vi "FlexMag - 23-03-2023.vi"() -> ()   [LabVIEW 2018] (continued)
                                n14725 = local write "pcgv4 auto open"(TRUE ("pcgv1 auto open")) -> ()
                                }
                                }
                              }
                            }
                          }
                          frame #1 {
                            n14726 = while {
                              i -> [w19971]
                              stop <- w19967 stop-if-true
                              n14727 = Greater Or Equal?(x=w19971, y=200) -> (x >= y?=w19973:bool)
                              n14728 = case shown="True" w19973 {
                                frame False {
                                }
                                frame True {
                                n14729 = local write "ch4 pumpdown error"(TRUE ("ch1 pumpdown error")) -> ()
                                n14730 = local write "Warning Message"("CH4 PumpDown process  is canceled !\nCH4 PC GV couldn't be opened" ("Warning Message")) -> ()
                                }
                              }
                              n14731 = local read "ch4 pumpdown alg"() -> (w19970:bool)
                              n14732 = local read "ch4_pcgv_gui"() -> (w19966:bool)
                              n14733 = local read "abort ch4"() -> (w19968:bool)
                              n14734 = Wait Until Next ms Multiple(millisecond multiple=u32 200) -> ()  [unwired: 1 out]
                              n14735 = Not(x=w19970) -> (.not. x?=w19969:bool)
                              n14736 = Compound Arithmetic op=OR(w19966, w19968, w19969) -> (w19967:bool)
                            }
                          }
                        }
                      }
                      frame True {
                      }
                    }
                  }
                }
              }
              frame #20 {
                n14737 = local read "ch4 pumpdown alg"() -> (w19976:bool)
                n14738 = case shown="True" w19976 {
                  frame False {
                  }
                  frame True {
                    n14739 = local read "abort ch4"() -> (w19977:bool)
                    n14740 = case shown="False" w19977 {
                      frame False {
                        n14741 = local write "ch4 pc gv open led"(TRUE ("ch1 ch vbv close")) -> ()
                        n14742 = Wait (ms)(milliseconds to wait=u32 1000) -> ()  [unwired: 1 out]
                      }
                      frame True {
                      }
                    }
                  }
                }
              }
              frame #21 {
                # "ch pressure check"
                n14743 = local read "ch4 pumpdown alg"() -> (w19980:bool)
                n14744 = case shown="True" w19980 {
                  frame False {
                  }
                  frame True {
                    n14745 = local read "abort ch4"() -> (w19981:bool)
                    n14746 = case shown="False" w19981 {
                      frame False {
                        n14747 = while {
                          i -> [w19988]
                          stop <- w19992 stop-if-true
                          # "30 min"
                          n14748 = Greater?(x=w19988, y=9000) -> (0:w19985:bool)
                          n14749 = case shown="True" w19985 {
                            frame False {
                            }
                            frame True {
                              n14750 = local write "Warning Message"("CH4 PumpDown process  is canceled !\nCH4 CH Pressure couldn't reach under 0.5 Torr" ("Warning Message")) -> ()
                              n14751 = local write "ch4 pumpdown error"(TRUE ("ch1 pumpdown error")) -> ()
                            }
                          }
                          n14752 = local read "ch4 ch pg torr"() -> (w19984:dbl)
                          n14753 = Less Or Equal?(x=w19984, y=0.5) -> (x <= y?=w19982:bool)
                          n14754 = case shown="False" w19982 {
                            tunnel: [FALSE TRUE] -> w19986
                            frame False {
                              n14755 = Wait Until Next ms Multiple(millisecond multiple=u32 200) -> ()  [unwired: 1 out]
                            }
                            frame True {
                            }
                          }
                          n14756 = local read "ch4 pumpdown alg"() -> (w19991:bool)
                          n14757 = local read "abort ch4"() -> (w19989:bool)
                          n14758 = Not(x=w19991) -> (.not. x?=w19990:bool)
                          n14759 = Compound Arithmetic op=OR(w19986, w19989, w19990) -> (w19992:bool)
                        }
                      }
                      frame True {
                      }
                    }
                  }
                }
              }
              frame #22 {
                n14760 = local read "ch4 pumpdown alg"() -> (w19998:bool)
                n14761 = case shown="True" w19998 {
                  frame False {
                  }
                  frame True {
                    n14762 = local read "abort ch4"() -> (w19999:bool)
                    n14763 = case shown="False" w19999 {
                      frame False {
                        n14764 = local write "ch4 ch press under 0.5 T led"(TRUE ("ch1 ch pressure led")) -> ()
                        n14765 = Wait (ms)(milliseconds to wait=u32 1000) -> ()  [unwired: 1 out]
                      }
                      frame True {
                      }
                    }
                  }
                }
              }
              frame #23 {
                # "ch 3 pressure check\nfor trns bp bv"
                n14766 = local read "ch4 pumpdown alg"() -> (w20002:bool)
                n14767 = case shown="True" w20002 {
                  frame False {
                  }
                  frame True {
                    n14768 = local read "abort ch4"() -> (w20003:bool)
                    n14769 = case shown="False" w20003 {
                      frame False {
                        n14770 = local read "ch3 ch pg torr"() -> (w20006:dbl)
                        n14771 = Less Or Equal?(x=w20006, y=0.5) -> (x <= y?=w20004:bool)
                        n14772 = case shown="True" w20004 {
                          frame False {
                          }
                          frame True {
                            n14773 = stacked-sequence {
                              frame #0 {
                                n14774 = while {
                                i -> [w20011]
                                stop <- w20015 stop-if-true
                                n14775 = Greater?(x=w20011, y=100) -> (0:w20008:bool)
                                n14776 = case shown="True" w20008 {
                                frame False {
                                }
                                frame True {
                                n14777 = local write "ch4 pumpdown error"(TRUE ("ch1 pumpdown error")) -> ()
                                n14778 = local write "Warning Message"("CH4 PumpDown process  is canceled !\nCH4 Trns BP Right couldn't be opened" ("Warning Message")) -> ()
                                }
                                }
                                n14779 = local read "CH4_Trns_BP_Right_DI"() -> (w20007:bool)
                                n14780 = case shown="False" w20007 {
                                tunnel: [FALSE TRUE] -> w20009
                                frame False {
                                n14781 = local write "CH4_Trns_BP_Right_DO"(TRUE ("CH1_Trns_BP_Left_DO")) -> ()
                                n14782 = Wait Until Next ms Multiple(millisecond multiple=u32 200) -> ()  [unwired: 1 out]
                                }
                                frame True {
                                }
                                }
                                n14783 = local read "ch4 pumpdown alg"() -> (w20014:bool)
                                n14784 = local read "abort ch4"() -> (w20012:bool)
                                n14785 = Not(x=w20014) -> (.not. x?=w20013:bool)
                                n14786 = Compound Arithmetic op=OR(w20009, w20012, w20013) -> (w20015:bool)
                                }
                              }
                              frame #1 {
                                n14787 = local read "ch4 pumpdown alg"() -> (w20022:bool)
                                n14788 = case shown="True" w20022 {
                                frame False {
                                }
                                frame True {
                                n14789 = local read "abort ch4"() -> (w20023:bool)
                                n14790 = case shown="False" w20023 {
                                frame False {
                                n14791 = local write "ch4 trns bp right open led"(TRUE ("ch1 tp start led")) -> ()
                                n14792 = Wait (ms)(milliseconds to wait=u32 1000) -> ()  [unwired: 1 out]
                                n14793 = local write "ch3_4 vacuum level"("VACUUM" ("ch3_4 vacuum level")) -> ()
                                }
                                frame True {
                                }
                                }
                                }
                                }
                              }
                              frame #2 {
                                n14794 = while {
                                i -> [w20029]
                                stop <- w20031 stop-if-true
                                n14795 = local read "ch4 pumpdown alg"() -> (w20032:bool)
                                n14796 = Wait Until Next ms Multiple(millisecond multiple=u32 200) -> ()  [unwired: 1 out]
                                n14797 = local read "abort ch4"() -> (w20034:bool)
                                n14798 = Greater?(x=w20029, y=100) -> (0:w20028:bool)
                                n14799 = Not(x=w20032) -> (.not. x?=w20033:bool)
                                n14800 = Compound Arithmetic op=OR(w20028, w20034, w20033) -> (w20031:bool)
                                }
                              }
                            }
                          }
                        }
                      }
                      frame True {
                      }
                    }
                  }
                }
              }
              frame #24 {
                # "ch pressure check"
                n14801 = local read "ch4 pumpdown alg"() -> (w20035:bool)
                n14802 = case shown="True" w20035 {
                  frame False {
                  }
                  frame True {
                    n14803 = local read "abort ch4"() -> (w20036:bool)
                    n14804 = case shown="False" w20036 {
                      frame False {
                        n14805 = while {
                          i -> [w20043]
                          stop <- w20047 stop-if-true
                          # "20 min"
                          n14806 = Greater?(x=w20043, y=6000) -> (0:w20040:bool)
                          n14807 = case shown="True" w20040 {
                            frame False {
                            }
                            frame True {
                              n14808 = local write "Warning Message"("CH4 PumpDown process  is canceled !\nCH4 CH Pressure couldn't  reach under 0.2 Torr" ("Warning Message")) -> ()
                              n14809 = local write "ch4 pumpdown error"(TRUE ("ch1 pumpdown error")) -> ()
                            }
                          }
                          n14810 = local read "ch4 ch pg torr"() -> (w20039:dbl)
                          n14811 = Less Or Equal?(x=w20039, y=0.2) -> (x <= y?=w20037:bool)
                          n14812 = case shown="True" w20037 {
                            tunnel: [FALSE TRUE] -> w20041
                            frame False {
                              n14813 = Wait Until Next ms Multiple(millisecond multiple=u32 200) -> ()  [unwired: 1 out]
                            }
                            frame True {
                            }
                          }
                          n14814 = local read "ch4 pumpdown alg"() -> (w20046:bool)
                          n14815 = local read "abort ch4"() -> (w20044:bool)
                          n14816 = Not(x=w20046) -> (.not. x?=w20045:bool)
                          n14817 = Compound Arithmetic op=OR(w20041, w20044, w20045) -> (w20047:bool)
                        }
                      }
                      frame True {
                      }
                    }
                  }
                }
              }
              frame #25 {
                # "tp start"
                n14818 = local read "ch4 pumpdown alg"() -> (w20053:bool)
                n14819 = case shown="True" w20053 {
                  frame False {
                  }
                  frame True {
                    n14820 = local read "abort ch4"() -> (w20054:bool)
                    n14821 = case shown="False" w20054 {
                      frame False {
                        n14822 = stacked-sequence {
                          frame #0 {
                            n14823 = flat-sequence {
                              frame #0 {
                                n14824 = local write "Tp4 auto start"(TRUE ("Tp1 auto start")) -> ()
                                n14825 = Wait (ms)(milliseconds to wait=u32 100) -> ()  [unwired: 1 out]
                              }
                              frame #1 {
                                n14826 = Wait (ms)(milliseconds to wait=u32 2000) -> ()  [unwired: 1 out]
                              }
                              frame #2 {
                                n14827 = disable-structure shown="Disabled" {
                                frame Disabled {
                                n14828 = local write "Tp1 Start initial"(TRUE ("Tp1 Start initial")) -> ()
                                }
                                frame Enabled {
                                }
                                }
                              }
                              frame #3 {
                                n14829 = Wait (ms)(milliseconds to wait=u32 2000) -> ()  [unwired: 1 out]
                              }
                              frame #4 {
                                n14830 = local write "Tp4 auto low speed"(TRUE ("Tp1 auto start")) -> ()
                                n14831 = Wait (ms)(milliseconds to wait=u32 100) -> ()  [unwired: 1 out]
                              }
                            }
                          }
                          frame #1 {
                            n14832 = while {
                              i -> [w20070]
                              stop <- w20064 stop-if-true
                              # "200 sec ?"
                              n14833 = Greater Or Equal?(x=w20070, y=1000) -> (x >= y?=w20063:bool)
                              n14834 = case shown="True" w20063 {
                                frame False {
                                }
                                frame True {
                                n14835 = local write "Warning Message"("CH4 PumpDown process  is canceled !\nCH4 TP couldn't be started" ("Warning Message")) -> ()
                                n14836 = local write "ch4 pumpdown error"(TRUE ("ch1 pumpdown error")) -> ()
                                }
                              }
                              n14837 = local read "ch4 pumpdown alg"() -> (w20067:bool)
                              n14838 = local read "ch4_tp_gui"() -> (w20062:bool)
                              n14839 = local read "abort ch4"() -> (w20065:bool)
                              n14840 = Not(x=w20067) -> (.not. x?=w20066:bool)
                              n14841 = Wait Until Next ms Multiple(millisecond multiple=u32 200) -> ()  [unwired: 1 out]
                              n14842 = Compound Arithmetic op=OR(w20062, w20065, w20066) -> (w20064:bool)
                            }
                          }
                        }
                      }
                      frame True {
                      }
                    }
                  }
                }
              }
              frame #26 {
                n14843 = local read "ch4 pumpdown alg"() -> (w20073:bool)
                n14844 = case shown="True" w20073 {
                  frame False {
                  }
                  frame True {
                    n14845 = local read "abort ch4"() -> (w20074:bool)
                    n14846 = case shown="False" w20074 {
                      frame False {
                        n14847 = local write "ch4 tp start led"(TRUE ("ch1 tp start led")) -> ()
                        n14848 = Wait (ms)(milliseconds to wait=u32 1000) -> ()  [unwired: 1 out]
                      }
                      frame True {
                      }
                    }
                  }
                }
              }
              frame #27 {
                n14849 = local read "ch4 pumpdown alg"() -> (w20077:bool)
                n14850 = case shown="True" w20077 {
                  frame False {
                  }
                  frame True {
                    n14851 = local read "abort ch4"() -> (w20078:bool)
                    n14852 = case shown="False" w20078 {
                      frame False {
                        n14853 = while {
                          i -> [w20085]
                          stop <- w20089 stop-if-true
                          # "30 min"
                          n14854 = Greater?(x=w20085, y=9000) -> (0:w20082:bool)
                          n14855 = case shown="True" w20082 {
                            frame False {
                            }
                            frame True {
                              n14856 = local write "Warning Message"("CH4 PumpDown process  is canceled !\nCH4 CH Pressure couldn't be reached under 0.01 Torr" ("Warning Message")) -> ()
                              n14857 = local write "ch4 pumpdown error"(TRUE ("ch1 pumpdown error")) -> ()
                            }
                          }
                          n14858 = local read "ch4 ch pg torr"() -> (w20081:dbl)
                          n14859 = Less Or Equal?(x=w20081, y=0.09) -> (x <= y?=w20079:bool)
                          n14860 = case shown="False" w20079 {
                            tunnel: [FALSE TRUE] -> w20083
                            frame False {
                              n14861 = Wait Until Next ms Multiple(millisecond multiple=u32 200) -> ()  [unwired: 1 out]
                            }
                            frame True {
                            }
                          }
                          n14862 = local read "ch4 pumpdown alg"() -> (w20088:bool)
                          n14863 = local read "abort ch4"() -> (w20086:bool)
                          n14864 = Not(x=w20088) -> (.not. x?=w20087:bool)
                          n14865 = Compound Arithmetic op=OR(w20083, w20086, w20087) -> (w20089:bool)
                        }
                      }
                      frame True {
                      }
                    }
                  }
                }
              }
              frame #28 {
                n14866 = local read "ch4 pumpdown alg"() -> (w20095:bool)
                n14867 = case shown="True" w20095 {
                  frame False {
                  }
                  frame True {
                    n14868 = local read "abort ch4"() -> (w20096:bool)
                    n14869 = case shown="False" w20096 {
                      frame False {
                        n14870 = local write "ch4 ch press under 0.01 T led"(TRUE ("ch1 pressure under 0.05 torr led")) -> ()
                        n14871 = Wait (ms)(milliseconds to wait=u32 1000) -> ()  [unwired: 1 out]
                      }
                      frame True {
                      }
                    }
                  }
                }
              }
              frame #29 {
                n14872 = local read "ch4 pumpdown alg"() -> (w20099:bool)
                n14873 = case shown="True" w20099 {
                  frame False {
                  }
                  frame True {
                    n14874 = local read "abort ch4"() -> (w20100:bool)
                    n14875 = case shown="False" w20100 {
                      frame False {
                        n14876 = stacked-sequence {
                          frame #0 {
                            n14877 = while {
                              i -> [w20105]
                              stop <- w20109 stop-if-true
                              n14878 = Greater?(x=w20105, y=200) -> (0:w20102:bool)
                              n14879 = case shown="True" w20102 {
                                frame False {
                                }
                                frame True {
                                n14880 = local write "Warning Message"("CH4 PumpDown process  is canceled !\nCH4 CC couldn't be opened" ("Warning Message")) -> ()
                                n14881 = local write "ch4 pumpdown error"(TRUE ("ch1 pumpdown error")) -> ()
                                }
                              }
                              n14882 = local read "CH4_CC_DI"() -> (w20101:bool)
                              n14883 = case shown="False" w20101 {
                                tunnel: [FALSE TRUE] -> w20103
                                frame False {
                                n14884 = Wait Until Next ms Multiple(millisecond multiple=u32 200) -> ()  [unwired: 1 out]
                                n14885 = local write "CH4_CC_DO"(TRUE ("CH1_CC_DO")) -> ()
                                }
                                frame True {
                                }
                              }
                              n14886 = local read "ch4 pumpdown alg"() -> (w20108:bool)
                              n14887 = local read "abort ch4"() -> (w20106:bool)
                              n14888 = Not(x=w20108) -> (.not. x?=w20107:bool)
                              n14889 = Compound Arithmetic op=OR(w20103, w20106, w20107) -> (w20109:bool)
                            }
                          }
                          frame #1 {
                            n14890 = while {
                              i -> [w20118]
                              stop <- w20120 stop-if-true
                              n14891 = local read "ch4 pumpdown alg"() -> (w20121:bool)
                              n14892 = local read "abort ch4"() -> (w20123:bool)
                              n14893 = Greater Or Equal?(x=w20118, y=300) -> (x >= y?=w20116:bool)
                              n14894 = Not(x=w20121) -> (.not. x?=w20122:bool)
                              n14895 = Compound Arithmetic op=OR(w20116, w20123, w20122) -> (w20120:bool)
                              n14896 = Wait Until Next ms Multiple(millisecond multiple=u32 200) -> ()  [unwired: 1 out]
                            }
                          }
                        }
                      }
                      frame True {
                      }
                    }
                  }
                }
              }
              frame #30 {
                n14897 = local read "ch4 pumpdown alg"() -> (w20124:bool)
                n14898 = case shown="True" w20124 {
                  frame False {
                  }
                  frame True {
                    n14899 = local read "abort ch4"() -> (w20125:bool)
                    n14900 = case shown="False" w20125 {
                      frame False {
                        n14901 = local write "ch4 cc open led"(TRUE ("ch1 ch cc open led")) -> ()
                        n14902 = Wait (ms)(milliseconds to wait=u32 1000) -> ()  [unwired: 1 out]
                      }
                      frame True {
                      }
                    }
                  }
                }
              }
              frame #31 {
                n14903 = local read "ch4 pumpdown alg"() -> (w20128:bool)
                n14904 = case shown="True" w20128 {
                  frame False {
                  }
                  frame True {
                    n14905 = local read "abort ch4"() -> (w20129:bool)
                    n14906 = case shown="False" w20129 {
                      frame False {
                        n14907 = while {
                          i -> [w20140]
                          stop <- w20144 stop-if-true
                          # "60 min"
                          n14908 = Multiply(x=27000 ("y"), y=3) -> (x*y=w20130:i32)
                          n14909 = Greater?(x=w20140, y=w20130) -> (0:w20138:bool)
                          n14910 = case shown="True" w20138 {
                            frame False {
                            }
                            frame True {
                              n14911 = local write "Warning Message"("CH4 PumpDown process  is canceled !\nCH4 CH Pressure couldn't reach to desired pressure" ("Warning Message")) -> ()
                              n14912 = local write "ch4 pumpdown error"(TRUE ("ch1 pumpdown error")) -> ()
                            }
                          }
                          n14913 = local read "ch4 cc torr"() -> (w20137:dbl)
                          n14914 = Multiply(x=0.75, y="ch4 desired pressure") -> (x*y=w20135:dbl)
                          n14915 = Less Or Equal?(x=w20137, y=w20135) -> (x <= y?=w20136:bool)
                          n14916 = case shown="True" w20136 {
                            tunnel: [FALSE TRUE] -> w20139
                            frame False {
                              n14917 = Wait Until Next ms Multiple(millisecond multiple=u32 200) -> ()  [unwired: 1 out]
                            }
                            frame True {
                            }
                          }
                          n14918 = local read "ch4 pumpdown alg"() -> (w20143:bool)
                          n14919 = local read "abort ch4"() -> (w20141:bool)
                          n14920 = Not(x=w20143) -> (.not. x?=w20142:bool)
                          n14921 = Compound Arithmetic op=OR(w20139, w20141, w20142) -> (w20144:bool)
                        }
                      }
                      frame True {
                      }
                    }
                  }
                }
              }
              frame #32 {
                n14922 = local read "ch4 pumpdown alg"() -> (w20150:bool)
                n14923 = case shown="True" w20150 {
                  frame False {
                  }
                  frame True {
                    n14924 = local read "abort ch4"() -> (w20151:bool)
                    n14925 = case shown="False" w20151 {
                      frame False {
                        n14926 = local write "ch4 desired pressure led"(TRUE ("ch1 pumdown completed led")) -> ()
                        n14927 = Wait (ms)(milliseconds to wait=u32 1000) -> ()  [unwired: 1 out]
                      }
                      frame True {
                      }
                    }
                  }
                }
              }
              frame #33 {
                n14928 = local read "ch4 pumpdown alg"() -> (w20154:bool)
                n14929 = case shown="True" w20154 {
                  frame False {
                  }
                  frame True {
                    n14930 = local read "abort ch4"() -> (w20155:bool)
                    n14931 = case shown="False" w20155 {
                      frame False {
                        w20157 = TRUE ("Buzzer DO")
                        n14932 = local write "Buzzer DO"(w20157) -> ()
                        n14933 = local write "ch4 pd completed led"(w20157) -> ()
                        n14934 = Wait (ms)(milliseconds to wait=u32 3000) -> ()  [unwired: 1 out]
                        n14935 = local write "CH4_BG_BV_DO"(TRUE ("CH1_BG_BV_DO")) -> ()
                        n14936 = local write "System Status"("CH4 PUMPDOWN PROCESS COMPLETED" ("System Status")) -> ()
                      }
                      frame True {
                      }
                    }
                  }
                }
              }
              frame #34 {
                n14937 = local read "ch4 pumpdown alg"() -> (w20160:bool)
                n14938 = case shown="True" w20160 {
                  frame False {
                  }
                  frame True {
                    n14939 = local read "abort ch4"() -> (w20161:bool)
                    n14940 = case shown="False" w20161 {
                      frame False {
                        w20163 = FALSE ("Buzzer DO")
                        n14941 = local write "Buzzer DO"(w20163) -> ()
                        n14942 = local write "ch4 pumpdown alg"(w20163) -> ()
                        n14943 = local write "Pump Down CH4"(w20163) -> ()
                        n14944 = Wait (ms)(milliseconds to wait=u32 3000) -> ()  [unwired: 1 out]
                        n14945 = local write "System Status"("SEMI-AUTOMATIC MODE " ("System Status")) -> ()
                      }
                      frame True {
                      }
                    }
                  }
                }
              }
            }
          }
          frame True {
          }
        }
      }
    }
    n14946 = case shown="True" "ch4 shutdown alg" {
      frame False {
      }
      frame True {
        n14947 = local read "abort ch4"() -> (w19384:bool)
        n14948 = case shown="False" w19384 {
          frame False {
            n14949 = stacked-sequence {
              frame #0 {
                n14950 = stacked-sequence {
                  frame #0 {
                    n14951 = local write "ch4 vent?"(FALSE ("ch1 vent?")) -> ()
                    n14952 = Wait (ms)(milliseconds to wait=u32 1000) -> ()  [unwired: 1 out]
                  }
                  frame #1 {
                    n14953 = local write "System Status"("CH4 SHUTDOWN PROCESS IN PROGRESS" ("System Status")) -> ()
                  }
                  frame #2 {
                    n14954 = Two Button Dialog(message="Do you want to Vent CH4 ?", 1:"No, SHUTDOWN only" ("F button name (\"Cancel\")"), 2:"Yes, VENT! CH4" ("T button name (\"OK\")")) -> (T button?=w19388:bool)
                    "ch4 vent?" <- w19388
                    n14955 = case shown="True" w19388 {
                      frame False {
                      }
                      frame True {
                        n14956 = local write "CH3_Trns_BP_Left_DO"(FALSE ("CH3_Trns_BP_Left_DO")) -> ()
                      }
                    }
                  }
                }
              }
              frame #1 {
                # "ATMs close"
                n14957 = local read "ch4 shutdown alg"() -> (w19393:bool)
                n14958 = case shown="True" w19393 {
                  frame False {
                  }
                  frame True {
                    n14959 = local read "abort ch4"() -> (w19394:bool)
                    n14960 = case shown="False" w19394 {
                      frame False {
                        w19395 = FALSE ("CH1_PL_ATM_DO")
                        n14961 = local write "CH4_PL_ATM_DO"(w19395) -> ()
                        n14962 = local write "CH4_CH_ATM_DO"(w19395) -> ()
                        n14963 = Wait (ms)(milliseconds to wait=u32 3000) -> ()  [unwired: 1 out]
                      }
                      frame True {
                      }
                    }
                  }
                }
              }
              frame #2 {
                n14964 = local read "ch4 shutdown alg"() -> (w19397:bool)
                n14965 = case shown="True" w19397 {
                  frame False {
                  }
                  frame True {
                    n14966 = local read "abort ch4"() -> (w19398:bool)
                    n14967 = case shown="False" w19398 {
                      frame False {
                        n14968 = local write "ch4 sd atms close led"(TRUE ("ch1 sd cc close led")) -> ()
                        n14969 = Wait (ms)(milliseconds to wait=u32 1000) -> ()  [unwired: 1 out]
                      }
                      frame True {
                      }
                    }
                  }
                }
              }
              frame #3 {
                # "CC close"
                n14970 = local read "ch4 shutdown alg"() -> (w19401:bool)
                n14971 = case shown="True" w19401 {
                  frame False {
                  }
                  frame True {
                    n14972 = local read "abort ch4"() -> (w19402:bool)
                    n14973 = case shown="False" w19402 {
                      frame False {
                        n14974 = while {
                          i -> [w19407]
                          stop <- w19411 stop-if-true
                          n14975 = Greater?(x=w19407, y=100) -> (0:w19404:bool)
                          n14976 = case shown="True" w19404 {
                            frame False {
                            }
                            frame True {
                              n14977 = local write "Warning Message"("CH4 ShutDown process  is canceled !\nCH4 CC couldn't be closed" ("Warning Message")) -> ()
                              n14978 = local write "ch4 shutdown error"(TRUE ("ch1 pumpdown error")) -> ()
                            }
                          }
                          n14979 = local read "CH4_CC_DI"() -> (w19403:bool)
                          n14980 = case shown="True" w19403 {
                            tunnel: [TRUE FALSE] -> w19405
                            frame False {
                            }
                            frame True {
                              n14981 = Wait Until Next ms Multiple(millisecond multiple=u32 200) -> ()  [unwired: 1 out]
                              n14982 = local write "CH4_CC_DO"(FALSE ("CH1_CC_DO")) -> ()
                            }
                          }
                          n14983 = local read "ch4 shutdown alg"() -> (w19410:bool)
                          n14984 = local read "abort ch4"() -> (w19408:bool)
                          n14985 = Not(x=w19410) -> (.not. x?=w19409:bool)
                          n14986 = Compound Arithmetic op=OR(w19405, w19408, w19409) -> (w19411:bool)
                        }
                      }
                      frame True {
                      }
                    }
                  }
                }
              }
              frame #4 {
                n14987 = local read "ch4 shutdown alg"() -> (w19418:bool)
                n14988 = case shown="True" w19418 {
                  frame False {
                  }
                  frame True {
                    n14989 = local read "abort ch4"() -> (w19419:bool)
                    n14990 = case shown="False" w19419 {
                      frame False {
                        n14991 = local write "ch4 sd cc close led"(TRUE ("ch1 sd cc close led")) -> ()
                        n14992 = Wait (ms)(milliseconds to wait=u32 1000) -> ()  [unwired: 1 out]
                      }
                      frame True {
                      }
                    }
                  }
                }
              }
              frame #5 {
                # "bg bv close"
                n14993 = local read "ch4 shutdown alg"() -> (w19422:bool)
                n14994 = case shown="True" w19422 {
                  frame False {
                  }
                  frame True {
                    n14995 = local read "abort ch4"() -> (w19423:bool)
                    n14996 = case shown="False" w19423 {
                      frame False {
                        n14997 = while {
                          i -> [w19428]
                          stop <- w19432 stop-if-true
                          n14998 = Greater?(x=w19428, y=100) -> (0:w19425:bool)
                          n14999 = case shown="True" w19425 {
                            frame False {
                            }
                            frame True {
                              n15000 = local write "Warning Message"("CH4 ShutDown process  is canceled !\nCH4 BG BV couldn't be closed" ("Warning Message")) -> ()
                              n15001 = local write "ch4 shutdown error"(TRUE ("ch1 pumpdown error")) -> ()
                            }
                          }
                          n15002 = local read "CH4_BG_BV_DI"() -> (w19424:bool)
                          n15003 = case shown="True" w19424 {
                            tunnel: [TRUE FALSE] -> w19426
                            frame False {
                            }
                            frame True {
                              n15004 = Wait Until Next ms Multiple(millisecond multiple=u32 200) -> ()  [unwired: 1 out]
                              n15005 = local write "CH4_BG_BV_DO"(FALSE ("CH1_CC_DO")) -> ()
                            }
                          }
                          n15006 = local read "ch4 shutdown alg"() -> (w19431:bool)
                          n15007 = local read "abort ch4"() -> (w19429:bool)
                          n15008 = Not(x=w19431) -> (.not. x?=w19430:bool)
                          n15009 = Compound Arithmetic op=OR(w19426, w19429, w19430) -> (w19432:bool)
                        }
                      }
                      frame True {
                      }
                    }
                  }
                }
              }
              frame #6 {
                n15010 = local read "ch4 shutdown alg"() -> (w19439:bool)
                n15011 = case shown="True" w19439 {
                  frame False {
                  }
                  frame True {
                    n15012 = local read "abort ch4"() -> (w19440:bool)
                    n15013 = case shown="False" w19440 {
                      frame False {
                        n15014 = local write "ch4 sd bg bv close led"(TRUE ("ch1 sd cc close led")) -> ()
                        n15015 = Wait (ms)(milliseconds to wait=u32 1000) -> ()  [unwired: 1 out]
                      }
                      frame True {
                      }
                    }
                  }
                }
              }
              frame #7 {
                # "TP stop"
                n15016 = local read "ch4 shutdown alg"() -> (w19443:bool)
                n15017 = case shown="True" w19443 {
                  frame False {
                  }
                  frame True {
                    n15018 = local read "abort ch4"() -> (w19444:bool)
                    n15019 = case shown="False" w19444 {
                      frame False {
                        n15020 = stacked-sequence {
                          frame #0 {
                            n15021 = flat-sequence {
                              frame #0 {
                                n15022 = local write "Tp4 auto stop"(TRUE ("Tp1 auto stop")) -> ()
                                n15023 = Wait (ms)(milliseconds to wait=u32 100) -> ()  [unwired: 1 out]
                              }
                              frame #1 {
                                n15024 = Wait (ms)(milliseconds to wait=u32 5000) -> ()  [unwired: 1 out]
                              }
                              frame #2 {
                                n15025 = local write "Tp4 auto stop"(TRUE ("Tp1 auto stop")) -> ()
                                n15026 = Wait (ms)(milliseconds to wait=u32 100) -> ()  [unwired: 1 out]
                              }
                            }
                          }
                          frame #1 {
                            n15027 = while {
                              i -> [w19461]
                              stop <- w19456 stop-if-true
                              n15028 = Multiply(x=3000 ("y"), y=5) -> (x*y=w19450:i32)
                              n15029 = Greater Or Equal?(x=w19461, y=w19450) -> (x >= y?=w19455:bool)
                              n15030 = case shown="True" w19455 {
                                frame False {
                                }
                                frame True {
                                n15031 = local write "Warning Message"("CH4 ShutDown process  is canceled !\nCH4 TP couldn't be stopped" ("Warning Message")) -> ()
                                n15032 = local write "ch4 shutdown error"(TRUE ("ch1 pumpdown error")) -> ()
                                }
                              }
                              n15033 = local read "ch4 shutdown alg"() -> (w19459:bool)
                              n15034 = local read "ch4_tp_gui"() -> (w19454:bool)
                              n15035 = local read "abort ch4"() -> (w19457:bool)
                              n15036 = Not(x=w19454) -> (.not. x?=w19453:bool)
                              n15037 = Not(x=w19459) -> (.not. x?=w19458:bool)
                              n15038 = Wait Until Next ms Multiple(millisecond multiple=u32 200) -> ()  [unwired: 1 out]
                              n15039 = Compound Arithmetic op=OR(w19453, w19457, w19458) -> (w19456:bool)
                            }
                          }
                        }
                      }
                      frame True {
                      }
                    }
                  }
                }
              }
              frame #8 {
                n15040 = local read "ch4 shutdown alg"() -> (w19464:bool)
                n15041 = case shown="True" w19464 {
                  frame False {
                  }
                  frame True {
                    n15042 = local read "abort ch4"() -> (w19465:bool)
                    n15043 = case shown="False" w19465 {
                      frame False {
                        n15044 = local write "ch4 sd tp stop led"(TRUE ("ch1 sd cc close led")) -> ()
                        n15045 = Wait (ms)(milliseconds to wait=u32 1000) -> ()  [unwired: 1 out]
                      }
                      frame True {
                      }
                    }
                  }
                }
              }
              frame #9 {
                # "tp bv close"
                n15046 = local read "ch4 shutdown alg"() -> (w19468:bool)
                n15047 = case shown="True" w19468 {
                  frame False {
                  }
                  frame True {
                    n15048 = local read "abort ch4"() -> (w19469:bool)
                    n15049 = case shown="False" w19469 {
                      frame False {
                        n15050 = while {
                          i -> [w19474]
                          stop <- w19478 stop-if-true
                          n15051 = Greater?(x=w19474, y=100) -> (0:w19471:bool)
                          n15052 = case shown="True" w19471 {
                            frame False {
                            }
                            frame True {
                              n15053 = local write "Warning Message"("CH4 ShutDown process  is canceled !\nCH4 TP BV couldn't be closed" ("Warning Message")) -> ()
                              n15054 = local write "ch4 shutdown error"(TRUE ("ch1 pumpdown error")) -> ()
                            }
                          }
                          n15055 = local read "CH4_TP_BV_DI"() -> (w19470:bool)
                          n15056 = case shown="True" w19470 {
                            tunnel: [TRUE FALSE] -> w19472
                            frame False {
                            }
                            frame True {
                              n15057 = Wait Until Next ms Multiple(millisecond multiple=u32 200) -> ()  [unwired: 1 out]
                              n15058 = local write "CH4_TP_BV_DO"(FALSE ("CH1_CC_DO")) -> ()
                            }
                          }
                          n15059 = local read "ch4 shutdown alg"() -> (w19477:bool)
                          n15060 = local read "abort ch4"() -> (w19475:bool)
                          n15061 = Not(x=w19477) -> (.not. x?=w19476:bool)
                          n15062 = Compound Arithmetic op=OR(w19472, w19475, w19476) -> (w19478:bool)
                        }
                      }
                      frame True {
                      }
                    }
                  }
                }
              }
              frame #10 {
                n15063 = local read "ch4 shutdown alg"() -> (w19485:bool)
                n15064 = case shown="True" w19485 {
                  frame False {
                  }
                  frame True {
                    n15065 = local read "abort ch4"() -> (w19486:bool)
                    n15066 = case shown="False" w19486 {
                      frame False {
                        n15067 = local write "ch4 sd tp bv close led"(TRUE ("ch1 sd cc close led")) -> ()
                        n15068 = Wait (ms)(milliseconds to wait=u32 1000) -> ()  [unwired: 1 out]
                      }
                      frame True {
                      }
                    }
                  }
                }
              }
              frame #11 {
                # "mp stop"
                n15069 = local read "ch4 shutdown alg"() -> (w19489:bool)
                n15070 = case shown="True" w19489 {
                  frame False {
                  }
                  frame True {
                    n15071 = local read "abort ch4"() -> (w19490:bool)
                    n15072 = case shown="False" w19490 {
                      frame False {
                        n15073 = while {
                          i -> [w19495]
                          stop <- w19499 stop-if-true
                          n15074 = Greater?(x=w19495, y=100) -> (0:w19492:bool)
                          n15075 = case shown="True" w19492 {
                            frame False {
                            }
                            frame True {
                              n15076 = local write "Warning Message"("CH4 ShutDown process  is canceled !\nCH4 MP couldn't be stopped" ("Warning Message")) -> ()
                              n15077 = local write "ch4 shutdown error"(TRUE ("ch1 pumpdown error")) -> ()
                            }
                          }
                          n15078 = local read "CH4_MP_DI"() -> (w19491:bool)
                          n15079 = case shown="True" w19491 {
                            tunnel: [TRUE FALSE] -> w19493
                            frame False {
                            }
                            frame True {
                              n15080 = Wait Until Next ms Multiple(millisecond multiple=u32 200) -> ()  [unwired: 1 out]
                              n15081 = local write "CH4_MP_DO"(FALSE ("CH1_CC_DO")) -> ()
                            }
                          }
                          n15082 = local read "ch4 shutdown alg"() -> (w19498:bool)
                          n15083 = local read "abort ch4"() -> (w19496:bool)
                          n15084 = Not(x=w19498) -> (.not. x?=w19497:bool)
                          n15085 = Compound Arithmetic op=OR(w19493, w19496, w19497) -> (w19499:bool)
                        }
                      }
                      frame True {
                      }
                    }
                  }
                }
              }
              frame #12 {
                n15086 = local read "ch4 shutdown alg"() -> (w19506:bool)
                n15087 = case shown="True" w19506 {
                  frame False {
                  }
                  frame True {
                    n15088 = local read "abort ch4"() -> (w19507:bool)
                    n15089 = case shown="False" w19507 {
                      frame False {
                        n15090 = local write "ch4 sd mp stop led"(TRUE ("ch1 sd cc close led")) -> ()
                        n15091 = Wait (ms)(milliseconds to wait=u32 1000) -> ()  [unwired: 1 out]
                      }
                      frame True {
                      }
                    }
                  }
                }
              }
              frame #13 {
                # "pl vbv open"
                n15092 = local read "ch4 shutdown alg"() -> (w19510:bool)
                n15093 = case shown="True" w19510 {
                  frame False {
                  }
                  frame True {
                    n15094 = local read "abort ch4"() -> (w19511:bool)
                    n15095 = case shown="False" w19511 {
                      frame False {
                        n15096 = while {
                          i -> [w19516]
                          stop <- w19520 stop-if-true
                          n15097 = Greater?(x=w19516, y=100) -> (0:w19513:bool)
                          n15098 = case shown="True" w19513 {
                            frame False {
                            }
                            frame True {
                              n15099 = local write "Warning Message"("CH4 ShutDown process  is canceled !\nCH4 PL VBV couldn't be opened" ("Warning Message")) -> ()
                              n15100 = local write "ch4 shutdown error"(TRUE ("ch1 pumpdown error")) -> ()
                            }
                          }
                          n15101 = local read "CH4_PL_VBV_DI"() -> (w19512:bool)
                          n15102 = case shown="False" w19512 {
                            tunnel: [FALSE TRUE] -> w19514
                            frame False {
                              n15103 = Wait Until Next ms Multiple(millisecond multiple=u32 200) -> ()  [unwired: 1 out]
                              n15104 = local write "CH4_PL_VBV_DO"(TRUE ("CH1_CC_DO")) -> ()
                            }
                            frame True {
                            }
                          }
                          n15105 = local read "ch4 shutdown alg"() -> (w19519:bool)
                          n15106 = local read "abort ch4"() -> (w19517:bool)
                          n15107 = Not(x=w19519) -> (.not. x?=w19518:bool)
                          n15108 = Compound Arithmetic op=OR(w19514, w19517, w19518) -> (w19520:bool)
                        }
                      }
                      frame True {
                      }
                    }
                  }
                }
              }
              frame #14 {
                n15109 = local read "ch4 shutdown alg"() -> (w19527:bool)
                n15110 = case shown="True" w19527 {
                  frame False {
                  }
                  frame True {
                    n15111 = local read "abort ch4"() -> (w19528:bool)
                    n15112 = case shown="False" w19528 {
                      frame False {
                        n15113 = local write "ch4 sd pl vbv open led"(TRUE ("ch1 sd cc close led")) -> ()
                        n15114 = Wait (ms)(milliseconds to wait=u32 1000) -> ()  [unwired: 1 out]
                      }
                      frame True {
                      }
                    }
                  }
                }
              }
              frame #15 {
                n15115 = local read "ch4 shutdown alg"() -> (w19531:bool)
                n15116 = case shown="True" w19531 {
                  frame False {
                  }
                  frame True {
                    n15117 = local read "abort ch4"() -> (w19532:bool)
                    n15118 = case shown="False" w19532 {
                      frame False {
                        n15119 = local read "ch4 vent?"() -> (w19533:bool)
                        n15120 = case shown="False" w19533 {
                          frame False {
                            n15121 = stacked-sequence {
                              frame #0 {
                                n15122 = local read "ch4 shutdown alg"() -> (w19534:bool)
                                n15123 = case shown="True" w19534 {
                                frame False {
                                }
                                frame True {
                                n15124 = flat-sequence {
                                frame #0 {
                                n15125 = local write "pcgv4 auto close"(TRUE ("pcgv1 auto open")) -> ()
                                }
                                frame #1 {
                                n15126 = Wait (ms)(milliseconds to wait=u32 2000) -> ()  [unwired: 1 out]
                                }
                                frame #2 {
                                n15127 = local write "pcgv4 auto close"(TRUE ("pcgv1 auto open")) -> ()
                                }
                                }
                                }
                                }
                              }
                              frame #1 {
                                n15128 = while {
                                i -> [w19545]
                                stop <- w19541 stop-if-true
                                n15129 = Greater Or Equal?(x=w19545, y=200) -> (x >= y?=w19547:bool)
                                n15130 = case shown="True" w19547 {
                                frame False {
                                }
                                frame True {
                                n15131 = local write "ch4 shutdown error"(TRUE ("ch1 pumpdown error")) -> ()
                                n15132 = local write "Warning Message"("CH4 ShutDown process  is canceled !\nCH4 PC GV couldn't be closed" ("Warning Message")) -> ()
                                }
                                }
                                n15133 = local read "ch4_pcgv_gui"() -> (w19538:bool)
                                n15134 = local read "abort ch4"() -> (w19542:bool)
                                n15135 = local read "ch4 shutdown alg"() -> (w19544:bool)
                                n15136 = Wait Until Next ms Multiple(millisecond multiple=u32 200) -> ()  [unwired: 1 out]
                                n15137 = Not(x=w19538) -> (.not. x?=w19539:bool)
                                n15138 = Not(x=w19544) -> (.not. x?=w19543:bool)
                                n15139 = Compound Arithmetic op=OR(w19539, w19542, w19543) -> (w19541:bool)
                                }
                              }
                            }
                          }
                          frame True {
                            n15140 = stacked-sequence {
                              frame #0 {
                                n15141 = local read "ch4 shutdown alg"() -> (w19550:bool)
                                n15142 = case shown="True" w19550 {
                                frame False {
                                }
                                frame True {
                                n15143 = flat-sequence {
                                frame #0 {
                                n15144 = local write "pcgv4 auto open"(TRUE ("pcgv1 auto open")) -> ()
                                }
                                frame #1 {
                                n15145 = Wait (ms)(milliseconds to wait=u32 2000) -> ()  [unwired: 1 out]
                                }
                                frame #2 {
                                n15146 = local write "pcgv4 auto open"(TRUE ("pcgv1 auto open")) -> ()
                                }
                                }
                                }
                                }
                              }
                              frame #1 {
                                n15147 = while {
                                i -> [w19560]
                                stop <- w19556 stop-if-true
                                n15148 = Greater Or Equal?(x=w19560, y=200) -> (x >= y?=w19562:bool)
                                n15149 = case shown="True" w19562 {
                                frame False {
                                }
                                frame True {
                                n15150 = local write "ch4 shutdown error"(TRUE ("ch1 pumpdown error")) -> ()
                                n15151 = local write "Warning Message"("CH4 ShutDown process  is canceled !\nCH4 PC GV couldn't be opened" ("Warning Message")) -> ()
                                }
                                }